vi "SMain.vi"() -> ()   [LabVIEW 2011] (continued)
          n194 = Equal?(x=w388, y="TRUE") -> ()  [unwired: 1 out]
          n195 = Equal?(x=w385, y="TRUE") -> (x = y?=w384:bool)
          n196 = local write "打印模式"(w347) -> ()
          n197 = case shown="\"N5224A\"" w396 {
            tunnel: [0 1 2] -> w395
            frame "E5071C", Default {
            }
            frame "N5230A(C)" {
            }
            frame "N5224A" {
            }
          }
          n198 = case shown="\"Dev3\"" w392 {
            tunnel: [0 1 2] -> w393
            frame "Dev1", Default {
            }
            frame "Dev2" {
            }
            frame "Dev3" {
            }
          }
          n199 = case shown="\"NI PCI-6509\", 默认" w394 {
            tunnel: [0 1] -> w350
            frame "NI PCI-6509", Default {
            }
            frame "LX MCU" {
            }
          }
          n200 = local write "Crosstalk  by Trace"(w372) -> ()
          n201 = local write "Local Database"(w384) -> ()
          n202 = local write "Dem 2X"(w368) -> ()
          n203 = local write "By Channel?"(w362) -> ()
          n204 = case shown="\"LUXSHARE - IIC\"" w344 {
            tunnel: [0 1] -> w346
            frame "RS232 - IIC", Default {
            }
            frame "LUXSHARE - IIC" {
            }
          }
          n205 = To Upper Case(1:w355) -> (0:w357:string)
          n206 = local write "RS232 I2C VISA"(w360) -> ()
          n207 = local write "VNA Model:"(w395) -> ()
          n208 = local write "Printer VISA"(w343) -> ()
          n209 = local write "DAQ  Model:"(w350) -> ()
          n210 = local write "DAQ Device"(w393) -> ()
          n211 = Equal?(x=w357, y="TRUE") -> (x = y?=w356:bool)
          n212 = local write "VISA COM"(w391) -> ()
          n213 = To Upper Case(1:w375) -> (0:w381:string)
          n214 = To Upper Case(1:w371) -> (0:w378:string)
          n215 = local write "upload"(w356) -> ()
          n216 = Equal?(x=w381, y="TRUE") -> (x = y?=w377:bool)
          n217 = Equal?(x=w378, y="TRUE") -> (x = y?=w376:bool)
          n218 = local write "Adaptor:"(w346) -> ()
          n219 = local write "Demo"(w377) -> ()
          n220 = local write "Manual"(w376) -> ()
          n221 = case shown="1" w350 {
            tunnel: [2 0] -> w352
            tunnel: [0 2] -> w351
            frame 0, Default {
            }
            frame 1 {
            }
          }
          n222 = disable-structure shown="禁用" {
            disable-tunnel: w356 -> [w401 _]
            frame Disabled {
              w402 = "Data UpLoad" ("项标识符")
              n223 = Current VI's Menubar() -> (w405:refnum<k9>)
              n224 = Get Menu Item Info(7:w402, 11:w405) -> (2:w403:string, 3:w404:refnum<k9>)  [unwired: 1 in, 5 out]
              n225 = Set Menu Item Info(6:w401, 7:w402, 9:TRUE ("已启用"), 10:w403, 11:w404) -> ()  [unwired: 2 in, 2 out]
            }
            frame Enabled {
            }
          }
          n226 = property on="DAQ Device" class="Ring (严格)"("DisabledEnum"=w351) -> ()  [unwired: 2 in, 2 out]
          n227 = property on="VISA COM" class="VISAName"("DisabledEnum"=w352) -> ()  [unwired: 2 in, 2 out]
          n228 = To Upper Case(1:w339) -> (0:w340:string)
          n229 = Equal?(x=w340, y="TRUE") -> (x = y?=w342:bool)
          n230 = local write "Use Counts?"(w342) -> ()
        }
      }
    }
    frame #4 {
      w441 = T8 {"Server"="", "DB"="", "PSW"="", "User"=""}  # DBSet
      n231 = call <vilib>:"Application Directory.vi"() -> ("Application Directory"=w498:path)
      n232 = Build Path(base path=w498, name or relative path="Database" ("名称或相对路径")) -> (appended path=w496:path)
      n233 = call <vilib>:"Application Directory.vi"() -> ("Application Directory"=w508:path)
      n234 = call <vilib>:"Application Directory.vi"() -> ("Application Directory"=w526:path)
      n235 = call <vilib>:"Check if File or Folder Exists.vi"("path"=w496) -> ("file or folder exists?"=w495:bool, "dup path"=w494:path)  [unwired: 8 in, 1 out]
      n236 = Build Path(base path=w526, name or relative path="EEPROM Code\\tempory_folder" ("名称或相对路径")) -> (appended path=w518:path)
      n237 = Build Path(base path=w508, name or relative path="Database" ("名称或相对路径")) -> (appended path=w506:path)
      n238 = case shown="假" w495 {
        tunnel: w494 -> [w555 w556]
        tunnel: [w554 w556] -> w493
        frame False {
          n239 = Create Folder(path (use dialog)=w555) -> (created path=w554:path)  [unwired: 2 in, 2 out]
        }
        frame True {
        }
      }
      n240 = call <vilib>:"Check if File or Folder Exists.vi"("path"=w518) -> ("file or folder exists?"=w517:bool, "dup path"=w516:path)  [unwired: 8 in, 1 out]
      n241 = call <vilib>:"Check if File or Folder Exists.vi"("path"=w506) -> ("file or folder exists?"=w505:bool, "dup path"=w504:path)  [unwired: 8 in, 1 out]
      n242 = case shown="假" w517 {
        tunnel: w516 -> [w579 w580]
        tunnel: [w578 w580] -> w515
        frame False {
          n243 = Create Folder(path (use dialog)=w579) -> (created path=w578:path)  [unwired: 2 in, 2 out]
        }
        frame True {
        }
      }
      n244 = case shown="假" w505 {
        tunnel: w504 -> [w574 w575]
        tunnel: [w573 w575] -> w503
        frame False {
          n245 = Create Folder(path (use dialog)=w574) -> (created path=w573:path)  [unwired: 2 in, 2 out]
        }
        frame True {
        }
      }
      n246 = Build Path(base path=w493, name or relative path="FigoConfig.xml" ("名称或相对路径")) -> (appended path=w491:path)
      n247 = call <vilib>:"Check if File or Folder Exists.vi"("path"=w491) -> ("file or folder exists?"=w490:bool, "dup path"=w466:path)  [unwired: 8 in, 1 out]
      n248 = call "deleteFolder_vna.vi"("input_path"=w515) -> ()  [unwired: 1 in]
      n249 = Build Path(base path=w503, name or relative path="DelayConfig.txt" ("名称或相对路径")) -> (appended path=w501:path)
      n250 = call <vilib>:"Check if File or Folder Exists.vi"("path"=w501) -> ("file or folder exists?"=w500:bool, "dup path"=w499:path)  [unwired: 8 in, 1 out]
      n251 = call <vilib>:"Application Directory.vi"() -> ("Application Directory"=w524:path)
      n252 = constructor class="CPLTSApplicationClass"() -> (reference out=w512:refnum<k24>)  [unwired: 3 in, 2 out]
      n253 = call "equipconfirm.vi"("path to XML document"=w466) -> ("确认结果"=w465:bool)
      n254 = Build Path(base path=w524, name or relative path="Database\\LabelList.xlsx" ("名称或相对路径")) -> (appended path=w522:path)
      n255 = call <vilib>:"Check if File or Folder Exists.vi"("path"=w522) -> ("error out"=w519:errorcluster, "file or folder exists?"=w521:bool, "dup path"=w520:path)  [unwired: 8 in]
      n256 = local read "打印模式"() -> (w511:enum16{"IT Print", "EE Print"})
      n257 = case shown="假" w465 {
        frame False {
          n258 = Quit LabVIEW(quit? (T)=TRUE ("退出？(T)")) -> ()
        }
        frame True {
        }
      }
      n259 = control-ref of="Test Status:"() -> (w422:refnum<vi>)
      n260 = case shown="真" w500 {
        tunnel: w499 -> [w561 w572]
        frame False {
          w557 = 100.0 ("写入延时（单位：ms）")
          w558 = 100.0 ("读取延时（单位：ms）")
          n261 = local write "读取延时（单位：ms）"(w558) -> ()
          n262 = global write "延时设置全局变量.vi" "写入延时"(w558) -> ()
          n263 = local write "Q写入延时（单位：ms）"(250.0 ("写入延时（单位：ms）")) -> ()
          n264 = local write "S写入延时（单位：ms）"(w557) -> ()
          n265 = global write "延时设置全局变量.vi" "写入延时"(w557) -> ()
          n266 = call-poly <vilib>:"Write To Spreadsheet File.vi"("2D data"=string[][] [["Q写入延时时间（ms）：", "250"], ["S写入延时时间（ms）：", "100"], ["读取延时时间（ms）：", "100"]], "file path (dialog if empty)"=w561) -> ()  [unwired: 6 in, 1 out]
        }
        frame True {
          n267 = call-poly <vilib>:"Read From Spreadsheet File.vi"("file path (dialog if empty)"=w572) -> ("all rows"=w571:string[][])  [unwired: 6 in, 4 out]
          n268 = Index Array(array=w571, index (col)=1 ("禁用的索引 (列)")) -> (element=w569:string[])  [unwired: 1 in]
          n269 = Index Array(array=w569, index #1=0 ("索引")) -> (element #1=w567:string, element #2=w565:string, element #3=w564:string)  [unwired: 2 in]
          n270 = Fract/Exp String To Number(string=w567) -> (number=w562:dbl)  [unwired: 3 in, 1 out]
          n271 = Fract/Exp String To Number(string=w564) -> (number=w566:dbl)  [unwired: 3 in, 1 out]
          n272 = Fract/Exp String To Number(string=w565) -> (number=w563:dbl)  [unwired: 3 in, 1 out]
          n273 = local write "Q写入延时（单位：ms）"(w562) -> ()
          n274 = global write "延时设置全局变量.vi" "写入延时"(w562) -> ()
          n275 = local write "S写入延时（单位：ms）"(w563) -> ()
          n276 = local write "读取延时（单位：ms）"(w566) -> ()
          n277 = global write "延时设置全局变量.vi" "读取延时"(w566) -> ()
        }
      }
      n278 = invoke class="CPLTSApplicationClass" method="ShowWindow"(reference=w512, "nCmdShow"="nCmdShow") -> (reference out=w514:refnum<k24>)  [unwired: 2 in, 3 out]
      n279 = case shown="\"IT Print\", 默认" w511 {
        frame "IT Print", Default {
          n280 = property on="MO:" class="Str"("Visible"=TRUE ("可见")) -> ()  [unwired: 2 in, 2 out]
        }
        frame "EE Print" {
          n281 = property on="MO:" class="Str"("Visible"=FALSE ("可见")) -> ()  [unwired: 2 in, 2 out]
        }
      }
      n282 = property on="属性节点" class="Str"(reference=w422, "Text.BGColor"=u32 16711680, "Text.TextColor"=u32 16448250) -> ()  [unwired: 1 in, 2 out]
      n283 = case shown="真" w490 {
        tunnel: w466 -> [_ w534]
        tunnel: [string[] ["net use \\\\172.200.20.86 Luxshare-ict /user:C040345", "\\\\172.20.20.86\\HuaweiData\\DataRoot\\XML", "net use \\\\172.20.20.113 mesuser /user:mesuser", "\\\\172.20.20.113\\emc\\HPTS\\VNA", "\\\\172.20.20.113\\emc\\HPTS\\SI", "false"] ("OutParaArray") w543] -> w489
        tunnel: [string[] ["false"] ("OutParaArray") w541] -> w472
        tunnel: ["A" ("node text") w537] -> w467
        tunnel: [string[] [] ("OutParaArray") w535] -> w451
        frame False {
        }
        frame True {
          w547 = "Mo" ("名称")
          w549 = "PN" ("名称")
          n284 = call "xmlConfigRead.vi"("path to XML document"=w534, "XPath expression"="//OtherPara/*") -> ("OutParaArray"=w541:string[])  [unwired: 2 out]
          n285 = call "xmlConfigRead.vi"("path to XML document"=w534, "XPath expression"="//UploadPara/*") -> ("OutParaArray"=w543:string[])  [unwired: 2 out]
          n286 = call "xmlConfigRead.vi"("path to XML document"=w534, "XPath expression"="//LastPartNo/*") -> ("OutParaVariant"=w551:variant)  [unwired: 2 out]
          n287 = call "xmlConfigRead.vi"("path to XML document"=w534, "XPath expression"="//LineID/Line/@Name") -> ("OutParaArray"=w532:string[])  [unwired: 2 out]
          n288 = call "xmlConfigRead.vi"("path to XML document"=w534, "XPath expression"="//DBSet/ConnectInfo/@*") -> ("OutParaArray"=w535:string[])  [unwired: 2 out]
          n289 = call "xmlConfigRead.vi"("path to XML document"=w534, "XPath expression"="//SystemList/CurrentNO/@Name") -> ("OutParaArray"=w539:string[])  [unwired: 2 out]
          n290 = Get Variant Attribute(Variant=w551, name=w549) -> (duplicate Variant=w552:variant, value=w550:variant)  [unwired: 2 in, 2 out]
          n291 = Get Variant Attribute(Variant=w552, name=w547) -> (value=w548:variant)  [unwired: 2 in, 3 out]
          n292 = property on="线别" class="Ring (严格)"("Strings []"=w532) -> ()  [unwired: 2 in, 2 out]
          n293 = Variant To Data(type=w547, Variant=w548) -> (data=w545:string)  [unwired: 1 in, 1 out]
          n294 = Variant To Data(type=w549, Variant=w550) -> (data=w546:string)  [unwired: 1 in, 1 out]
          n295 = property on="P/N:" class="Str"("Val(Sgnl)"=w546) -> ()  [unwired: 2 in, 2 out]
          n296 = local write "MO:"(w545) -> ()
          n297 = Index Array(array=w539, index=0 ("索引")) -> (element=w537:string)
        }
      }
      "SystemMode" <- w467
      n298 = case shown="假" w521 {
        tunnel: w520 -> [w584 _]
        tunnel: w519 -> [_ _]
        frame False {
          n299 = call <vilib>:"New Report.vi"("report type"=T16."Excel") -> ("report out"=w586:refnum<class "NI_report.lvclass">)  [unwired: 13 in, 1 out]
          n300 = call <vilib>:"Excel Get Worksheet.vi"("report in"=w586, "worksheet index (0)"=0) -> ("report out"=w588:refnum<class "NI_report.lvclass">, "error out"=w587:errorcluster)  [unwired: 12 in]
          n301 = Build Array(string[] ["料号", "日期类型", "年份起始位", "年份结束位", "周起始位", "周结束位", "月份起始位", "月份结束位", "天数起始位", "天数结束位", "流水号起始位", "流水号起始位"]) -> (w581:string[][])
          n302 = call-poly <vilib>:"Excel Easy Table.vi"("report in"=w588, "text data"=w581, "error in (no error)"=w587) -> ("report out"=w583:refnum<class "NI_report.lvclass">)  [unwired: 8 in, 4 out]
          n303 = call-dynamic "Save Report to File.vi"("report in"=w583, "report file path"=w584) -> ("report out"=w591:refnum<class "NI_report.lvclass">, "error out"=w590:errorcluster)  [unwired: 12 in]
          n304 = call-dynamic "Dispose Report.vi"("report in"=w591, "wait until printing completed? (T)"=TRUE, "error in (no error)"=w590) -> ()  [unwired: 12 in, 1 out]
        }
        frame True {
        }
      }
      n305 = local write "Excel?"(TRUE ("Excel?")) -> ()
      n306 = local write "upload"(TRUE ("upload")) -> ()
      n307 = invoke class="CPLTSApplicationClass" method="CloseAllFiles"(reference=w514) -> ()  [unwired: 2 in, 3 out]
      n308 = constructor class="LabelPrintHelper"() -> (reference out=→"PRINT":refnum<k24>)  [unwired: 3 in, 2 out]
      n309 = constructor class="MESDataServices"() -> (reference out=→"SN":refnum<k24>)  [unwired: 3 in, 2 out]
      n310 = Delete From Array(array=w451, length=4 ("长度")) -> (deleted portion=w442:string[], array with subset deleted=w450:string[])  [unwired: 1 in]
      n311 = Index Array(array=w450) -> (element #1=w449:string, element #2=w448:string, element #3=w446:string, element #4=w447:string)  [unwired: 4 in]
      n312 = global write "全局.vi" "print templete"(FALSE ("print templete")) -> ()
      n313 = call "DES.vi"("sourceData"=w446, "操作"=enum16{"DES_Encrypt", "DES_Decrypt"}."DES_Decrypt") -> ("加密后字符串"=w445:string)  [unwired: 8 in, 1 out]
      n314 = Index Array(array=w472, index #1=0 ("索引"), index #2=1 ("索引"), index #3=2 ("索引"), index #4=3 ("索引")) -> (element #1=w469:string, element #2=w462:string, element #3=w458:string, element #4=w453:string)
      n315 = Decimal String To Number(string=w453) -> (number=→"startSN":i32)  [unwired: 2 in, 1 out]
      n316 = Bundle By Name(cluster=w441, "Server"=w449, "DB"=w448, "PSW"=w445, "User"=w447) -> (→"DB1":T8)
      n317 = Decimal String To Number(string=w462) -> (number=w461:i32)  [unwired: 2 in, 1 out]
      n318 = Equal?(x=w469, y="true") -> (x = y?=→"ConvertStyle":bool)
      n319 = Index Array(array=w489, index #1=0 ("索引"), index #2=1 ("索引"), index #3=2 ("索引"), index #4=3 ("索引"), index #5=4 ("索引"), index #6=5 ("索引"), index #7=6 ("索引"), index #8=7 ("索引"), index #9=8 ("索引")) -> (element #1=→"NetCmd":string, element #2=→"NetPathHW":string, element #3=→"NetCmdCompress":string, element #4=w481:string, element #5=w480:string, element #6=w476:string, element #7=w428:string, element #8=→"NetTemppath":string, element #9=→"NetLocalpath":string)
      n320 = String To Path(string=w481) -> (path=→"NetPathCompress1":path)
      n321 = String To Path(string=w480) -> (path=→"NetPathCompress2":path)
      n322 = Equal?(x=w458, y="true") -> (x = y?=→"TestResultSave":bool)
      n323 = global write "全局.vi" "logsetting"(w461) -> ()
      n324 = Equal?(x=w476, y="true") -> (x = y?=→"AlarmDisplay":bool)
      n325 = Index Array(array=w442) -> (element #1=w440:string, element #2=w439:string, element #3=w437:string, element #4=w435:string)  [unwired: 4 in]
      n326 = call "DES.vi"("sourceData"=w437, "操作"=enum16{"DES_Encrypt", "DES_Decrypt"}."DES_Decrypt") -> ("加密后字符串"=w438:string)  [unwired: 8 in, 1 out]
      n327 = Equal?(x=w428, y="true") -> (x = y?=→"asychronus":bool)
      n328 = Bundle By Name(cluster=w441, "Server"=w440, "DB"=w439, "PSW"=w438, "User"=w435) -> (→"DB2":T8)
    }
    frame #5 {
      n329 = control-ref of="Test Status:"() -> (w593:refnum<vi>)
      n330 = global write "全局.vi" "Test Status"(w593) -> ()
      n331 = property on="Type" class="Ring (严格)"("Val(Sgnl)"=u16 0 ("值(信号)")) -> ()  [unwired: 2 in, 2 out]
      n332 = property on="Start Test" class="Bool"("BoolText.Text"="START TEST" ("布尔文本.文本")) -> ()  [unwired: 2 in, 2 out]
      n333 = local write "caliDataSelect"(FALSE ("caliDataSelect")) -> ()
    }
    frame #6 {
      n334 = while {
        tunnel: [w599] -> _
        stop <- w599 stop-if-true
        n335 = case shown="\"wait\", 默认" "State" {
          tunnel: [_ _ TRUE ("Stop") w1882] -> w599
          frame "test" {
            n336 = stacked-sequence {
              frame #0 {
                n337 = property on="Start Test" class="Bool"("DisabledEnum"=2) -> ()  [unwired: 2 in, 2 out]
                n338 = local write "proBar"(u8 0 ("proBar")) -> ()
                n339 = local write "preStation"("" ("preStation")) -> ()
                n340 = property on="preStation" class="Str"("Visible"=FALSE ("可见")) -> ()  [unwired: 2 in, 2 out]
                n341 = control-ref of="Test Status:"() -> (w601:refnum<vi>)
                n342 = property on="属性节点" class="Str"(reference=w601, "Text.BGColor"=u32 16448250, "Text.TextColor"=u32 0) -> ()  [unwired: 1 in, 2 out]
                n343 = property on="S/N:" class="Str"("DisabledEnum"=T17."Disabled and Grayed Out" ("禁用")) -> ()  [unwired: 2 in, 2 out]
                n344 = local write "strFSN 原始SN"("" ("strFSN 原始SN")) -> ()
                n345 = local write "Current Testing Label/当前测试条码"("") -> ()
                n346 = local write "midVar_time_date"(timestamp(3534465477 s since 1904-01-01) ("midVar_time_date")) -> ()
                n347 = local write "未经进制转换的sn(客户 jin zhi sn)"("" ("未经进制转换的sn(客户 jin zhi sn)")) -> ()
                n348 = local write "Test Status:"("" ("Test Status:")) -> ()
                n349 = local write "要烧录的DateCode"("" ("要烧录的DateCode")) -> ()
                n350 = local write "要烧录的时间和Sn"("" ("要烧录的时间和Sn")) -> ()
                "customer date" <- "" ("customer date")
                "Shi jin zhi sn" <- "" ("Shi jin zhi sn")
              }
              frame #1 {
                n351 = local read "Use Counts?"() -> (w619:bool)
                n352 = case shown="真" w619 {
                  tunnel: [TRUE w622] -> w618
                  frame False {
                  }
                  frame True {
                    n353 = local read "RS232 I2C Counts"() -> (w625:refnum<visa-resource-name>)
                    n354 = call "读取.vi"("RS232 I2C Counts"=w625) -> ("result"=w622:bool, "UseAge"=w623:i64, "Used"=w624:i64)  [unwired: 8 in]
                    n355 = local write "Used"(w624) -> ()
                    n356 = local write "UseAge"(w623) -> ()
                  }
                }
                n357 = local write "test time"(string[] [] ("test time")) -> ()
                n358 = case shown="真" w618 {
                  frame False {
                    # "测试版使用次数是否合格"
                    n359 = local read "UseAge"() -> (w630:i64)
                    n360 = local read "Used"() -> (w633:i64)
                    n361 = local write "Go"(FALSE ("Go")) -> ()
                    n362 = Number To Decimal String(number=w633) -> (decimal integer string=w632:string)  [unwired: 1 in]
                    n363 = Number To Decimal String(number=w630) -> (decimal integer string=w629:string)  [unwired: 1 in]
                    n364 = Concatenate Strings("测试板使用了", w632, "次,超过了最大使用寿命:" ("字符串"), w629, "不允许继续使用，请更换测试板后继续测试！" ("字符串"), "或者修改使用次数的动作失败！" ("字符串")) -> (w627:string)
                    n365 = One Button Dialog(message=w627) -> ()  [unwired: 1 in, 1 out]
                  }
                  frame True {
                    # "测试版使用次数是否合格"
                    n366 = local read "线别确认"() -> (w637:bool)
                    n367 = Not(x=w637) -> (.not. x?=w636:bool)
                    n368 = case shown="假" w636 {
                      frame False {
                        n369 = local read "DateCode8Value_0X30"() -> (w639:i32)
                        n370 = local read "打印模式"() -> (w642:enum16{"IT Print", "EE Print"})
                        n371 = local read "AutoSN"() -> (w643:bool)
                        n372 = local read "ConvertStyle"() -> (w641:bool)
                        n373 = Format Into String(initial string="当前datacode为:0X", w639) -> (resulting string=w638:string)  [unwired: 2 in, 1 out]
                        n374 = call "addStatus.vi"("msg"=w638) -> ()  [unwired: 10 in, 1 out]
                        n375 = case shown="假" w643 {
                          tunnel: w642 -> [_ w700]
                          tunnel: w641 -> [w653 w699]
                          tunnel: w639 -> [w652 w698]
                          frame False {
                            # "前站数据是否需要管控"
                            n376 = local read "S/N:"() -> (w650:string)
                            n377 = local read "P/N:"() -> (w645:string)
                            n378 = local read "DB1"() -> (w649:T8)
                            n379 = call "前站查询(T1).vi"("Station"="preStation", "Pre Check"="Pre Check", "PN"=w645, "DBSet"=w649, "SN"=w650) -> ("判定"=w648:bool)  [unwired: 6 in]
                            n380 = call "前站查询.vi"("DBSet"=w649, "SN"=w650) -> ("判定"=w647:bool)  [unwired: 9 in]
                            n381 = And(x=w647, y=w648) -> (x .and. y?=w646:bool)
                            n382 = case shown="真" w646 {
                              tunnel: w653 -> [_ w657]
                              tunnel: w652 -> [_ w656]
                              frame False {
                                n383 = One Button Dialog(message="前面有不良维修记录待处理，请进行处理后再测试" ("消息")) -> ()  [unwired: 1 in, 1 out]
                                n384 = local write "Go"(FALSE ("Go")) -> ()
                              }
                              frame True {
                                n385 = stacked-sequence {
                                tunnel: w657 -> [_ w665]
                                tunnel: w656 -> [_ w664]
                                frame #0 {
                                n386 = local read "DB1"() -> (w658:T8)
                                n387 = local read "LastSN"() -> (w662:string)
                                n388 = local read "S/N:"() -> (w661:string)
                                n389 = call "重测.vi"("Last SN"=w662, "DBSet"=w658, "SN"=w661) -> ("继续?"=→"继续?":bool, "重测原因"=→"重测原因":string)  [unwired: 6 in, 1 out]
                                }
                                frame #1 {
                                n390 = local read "继续?"() -> (w663:bool)
                                n391 = case shown="真" w663 {
                                tunnel: w665 -> [_ w677]
                                tunnel: w664 -> [_ w676]
                                frame False {
                                n392 = local write "Go"(FALSE ("Go")) -> ()
                                }
                                frame True {
                                # "20160919增加从labelprint表查询，理由：作业流程变更，第一站就打条码。"
                                # "针对重工已经打印标签\n的进行修改，从资讯\n数据库中查到SN对应\n的信息回来进行测试"
                                n393 = local read "DB1"() -> (w674:T8)
                                n394 = local read "P/N:"() -> (w696:string)
                                n395 = local read "Local Database"() -> (w668:bool)
                                n396 = local read "mid_str_labelType"() -> (w694:string)
                                n397 = local read "labelConfig"() -> (w693:string[])
                                n398 = local read "打印模式"() -> (w671:enum16{"IT Print", "EE Print"})
                                n399 = local read "校验信息"() -> (w673:T7)
                                n400 = Equal?(x=w671, y=enum16{"IT Print", "EE Print"}."EE Print") -> (x = y?=w669:bool)
                                n401 = Or(x=w668, y=w669) -> (x .or. y?=w667:bool)
                                n402 = local read "S/N:"() -> (w695:string)
                                "LastSN" <- w695
                                n403 = local read "mid_array_eep"() -> (w692:string[][])
                                n404 = call "精简框图4.vi"("P/N:"=w696, "mid_str_labelType"=w694, "DateCode8Value_0X30"=w676, "Convert Style"=w677, "LocalDataBase?"=w667, "labelConfig"=w693, "mid_array_eep"=w692, "SNKeep"="SN Keep", "S/N"=w695, "DBSet"=w674, "校验信息"=w673) -> ("show_date"=w681:timestamp, "要烧录的时间和Sn"=w691:string, "未经进制转换的sn(客户 jin zhi sn)"=w682:string, "要烧录的DateCode"=w690:string, "strFSN 原始 Customer sn"=w683:string, "输出的label内容"=w680:string, "Go"=w679:bool, "mid_array_temp_int"=w689:u8[][], "S/N:"=w688:string, "Customer Date"=w687:string, "shi jin zhi sn"=w686:string, "Report No."=w685:string, "Sample #"=w684:string)  [unwired: 4 in]
                                n405 = And(x=w679, y=TRUE) -> (x .and. y?=w678:bool)
                                n406 = local write "Go"(w678) -> ()
                                n407 = local write "midVar_time_date"(w681) -> ()
                                n408 = local write "strFSN 原始SN"(w683) -> ()
                                n409 = local write "未经进制转换的sn(客户 jin zhi sn)"(w682) -> ()
                                n410 = local write "要烧录的时间和Sn"(w691) -> ()
                                n411 = local write "要烧录的DateCode"(w690) -> ()
                                n412 = local write "Current Testing Label/当前测试条码"(w680) -> ()
                                n413 = local write "mid_array_temp_int"(w689) -> ()
                                n414 = local write "S/N:"(w688) -> ()
                                n415 = local write "customer date"(w687) -> ()
                                n416 = local write "Shi jin zhi sn"(w686) -> ()
                                n417 = local write "Report No."(w685) -> ()
                                n418 = local write "Sample #"(w684) -> ()
                                n419 = local write "midVar_str_SN"(w680) -> ()
                                }
                                }
                                }
                                }
                              }
                            }
                          }
                          frame True {
                            n420 = local write "重测原因"("firsttest" ("重测原因")) -> ()
                            n421 = case shown="\"IT Print\", 默认" w700 {
                              tunnel: w699 -> [w704 w733]
                              tunnel: w698 -> [w702 w727]
                              frame "IT Print", Default {
                                # "没有转进制的流水"
                                # "mid_array_temp_int 是展开后的烧录文件"
                                # "通过MIS获得Sn"
                                n422 = local read "MO:"() -> (w713:string)
                                n423 = local read "mid_str_labelType"() -> (w721:string)
                                n424 = local read "SN"() -> (w703:refnum<k24>)
                                n425 = local read "labelConfig"() -> (w720:string[])
                                n426 = local read "mid_array_eep"() -> (w719:string[][])
                                n427 = local read "P/N:"() -> (w722:string)
                                n428 = local read "校验信息"() -> (w701:T7)
                                n429 = call "精简框图3.vi"("P/N:"=w722, "mid_str_labelType"=w721, "DateCode8Value_0X30"=w702, "Convert Style"=w704, "新引用"=w703, "labelConfig"=w720, "mid_array_eep"=w719, "工单号"=w713, "校验信息"=w701) -> ("show_date"=w712:timestamp, "要烧录的时间和Sn"=→"要烧录的时间和Sn":string, "未经进制转换的sn(客户 jin zhi sn)"=w705:string, "要烧录的DateCode"=→"要烧录的DateCode":string, "strFSN 原始 Customer sn"=w708:string, "输出的label内容"=w711:string, "Go"=w714:bool, "mid_array_temp_int"=w718:u8[][], "S/N:"=w717:string, "Customer Date"=w707:string, "shi jin zhi sn"=w706:string, "Report No."=w716:string, "Sample #"=w715:string)  [unwired: 6 in]
                                "Current Testing Label/当前测试条码" <- w711
                                n430 = local write "mid_array_temp_int"(w718) -> ()
                                n431 = local write "S/N:"(w717) -> ()
                                n432 = local write "Report No."(w716) -> ()
                                n433 = local write "Sample #"(w715) -> ()
                                n434 = local write "midVar_str_SN"(w711) -> ()
                                n435 = local write "Go"(w714) -> ()
                                n436 = local write "midVar_time_date"(w712) -> ()
                                n437 = local write "未经进制转换的sn(客户 jin zhi sn)"(w705) -> ()
                                n438 = local write "strFSN 原始SN"(w708) -> ()
                                n439 = local write "customer date"(w707) -> ()
                                n440 = local write "Shi jin zhi sn"(w706) -> ()
                              }
                              frame "EE Print" {
                                n441 = local read "startSN"() -> (w724:i32)
                                n442 = control-ref of="Test Status:"() -> (w731:refnum<vi>)
                                n443 = local read "mid_str_labelType"() -> (w737:string)
                                n444 = local read "mid_str_snformat"() -> (w736:string)
                                n445 = local read "P/N:"() -> (w734:string)
                                n446 = local read "mid_array_eep"() -> (w732:string[][])
                                n447 = local read "校验信息"() -> (w723:T7)
                                n448 = property class="Str"(reference=w731) -> (reference out=w729:refnum<vi>, "Value"=w730:string)  [unwired: 1 in, 1 out]
                                n449 = call "精简框图1.vi"("mid_str_labelType"=w737, "mid_array_eep"=w732, "mid_str_snformat"=w736, "Convert Style"=w733, "DateCode8Value_0X30"=w727, "P/N"=w734, "Sart SN"=w724, "校验信息"=w723) -> ("LocalSN Generate Status"=w726:string, "midVar_time_date"=w738:timestamp, "midVar_str_SN"=w739:string, "mid_array_temp_int"=w740:u8[][], "S/N:"=w741:string, "Report No."=w742:string, "Sample #"=w743:string)  [unwired: 5 in]
                                n450 = Concatenate Strings(w730, "\n", w726) -> (w728:string)
                                n451 = local write "Go"(TRUE ("Go")) -> ()
                                n452 = local write "midVar_time_date"(w738) -> ()
                                n453 = local write "midVar_str_SN"(w739) -> ()
                                n454 = local write "mid_array_temp_int"(w740) -> ()
                                n455 = local write "S/N:"(w741) -> ()
                                n456 = local write "Report No."(w742) -> ()
                                n457 = local write "Sample #"(w743) -> ()
                                n458 = property class="Str"(reference=w729, "Value"=w728) -> ()  [unwired: 1 in, 2 out]
                              }
                            }
                          }
                        }
                      }
                      frame True {
                        n459 = local write "Go"(FALSE ("Go")) -> ()
                        n460 = One Button Dialog(message="线别未确认" ("消息")) -> ()  [unwired: 1 in, 1 out]
                      }
                    }
                  }
                }
              }
              frame #2 {
                n461 = local read "Go"() -> (w746:bool)
                n462 = case shown="真" w746 {
                  frame False {
                    w750 = 0
                    n463 = property on="S/N:" class="Str"("Key Focus"=TRUE ("键选中")) -> ()  [unwired: 2 in, 2 out]
                    n464 = local write "State"("wait" ("state")) -> ()
                    n465 = local write "S/N:"("") -> ()
                    n466 = property on="S/N:" class="Str"("DisabledEnum"=T17."Enabled" ("禁用")) -> ()  [unwired: 2 in, 2 out]
                    n467 = property on="Start Test" class="Bool"("DisabledEnum"=w750) -> ()  [unwired: 2 in, 2 out]
                    n468 = property on="Tab_Graph" class="TabCtl (严格)"("Value"=w750) -> ()  [unwired: 2 in, 2 out]
                  }
                  frame True {
                    n469 = local read "P/N:"() -> (w756:string)
                    n470 = local read "VNA Model:"() -> (w762:enum16{"E5071C", "N5230A(C)", "N5224A"})
                    n471 = local read "Spec _Col"() -> (w757:i32[])
                    n472 = control-ref of="Test Status:"() -> (w761:refnum<vi>)
                    n473 = local read "VNA VISA"() -> (w763:refnum<visa-resource-name>)
                    n474 = local read "S/N:"() -> (w760:string)
                    n475 = call "Sample name judge.vi"("Sample  Name:"=w756, "START input"=TRUE) -> ("START output"=w764:bool)
                    n476 = case shown="真" w764 {
                      tunnel: "DAQ Device" -> [_ w784]
                      tunnel: w763 -> [_ w783]
                      tunnel: w762 -> [_ w782]
                      tunnel: w761 -> [_ w781]
                      tunnel: w760 -> [_ w780]
                      tunnel: "Port Type" -> [_ w779]
                      tunnel: "Demo" -> [_ w778]
                      tunnel: w757 -> [_ w777]
                      tunnel: w756 -> [_ w776]
                      tunnel: "Manual" -> [_ w775]
                      tunnel: "VISA COM" -> [_ w774]
                      tunnel: "DAQ  Model:" -> [_ w773]
                      tunnel: "Crosstalk  by Trace" -> [_ w772]
                      frame False {
                        w771 = 0
                        n477 = property on="S/N:" class="Str"("Key Focus"=TRUE ("键选中")) -> ()  [unwired: 2 in, 2 out]
                        n478 = local write "State"("wait" ("state")) -> ()
                        n479 = local write "S/N:"("") -> ()
                        n480 = property on="Start Test" class="Bool"("DisabledEnum"=w771) -> ()  [unwired: 2 in, 2 out]
                        n481 = property on="S/N:" class="Str"("DisabledEnum"=T17."Enabled" ("禁用")) -> ()  [unwired: 2 in, 2 out]
                        n482 = property on="Tab_Graph" class="TabCtl (严格)"("Value"=w771) -> ()  [unwired: 2 in, 2 out]
                      }
                      frame True {
                        n483 = stacked-sequence {
                          seq-local: [_ _ _ _ _ _ _ _ _ _ w1439 _ _ _ _ _ _] -> [_ _ _ _ _ _ _ _ _ _ _ w1464 _ _ _ _ _]
                          tunnel: w784 -> [_ _ _ w925 w1066 w1161 _ _ _ _ _ w1483 _ _ _ _ _]
                          tunnel: w783 -> [_ _ _ w924 w1065 w1160 _ _ _ _ _ _ _ _ _ _ _]
                          tunnel: w782 -> [_ _ _ w923 w1064 w1159 _ _ _ _ _ _ _ _ _ _ _]
                          tunnel: w776 -> [_ _ w868 w922 w1063 w1158 _ _ _ _ _ _ _ _ _ _ _]
                          tunnel: w781 -> [_ _ w849 w921 w1062 w1157 _ _ w1281 w1345 w1441 w1481 w1531 _ w1727 _ _]
                          tunnel: w780 -> [_ _ w860 w920 w1061 w1156 _ _ _ _ _ _ _ _ _ _ _]
                          tunnel: w779 -> [_ _ _ w914 w1059 w1154 _ _ _ _ _ _ _ _ _ _ _]
                          tunnel: w778 -> [_ _ _ w904 w1049 w1144 _ w1261 _ w1343 _ w1476 _ _ w1722 w1778 _]
                          tunnel: w777 -> [_ _ _ w913 w1060 w1155 _ _ _ _ _ _ _ _ _ _ _]
                          tunnel: w775 -> [_ _ _ w903 w1048 w1143 _ _ _ _ _ w1477 _ _ _ _ _]
                          tunnel: w774 -> [_ _ _ w909 w1055 w1149 _ _ _ _ _ w1474 _ _ _ _ _]
                          tunnel: w773 -> [_ _ _ w908 w1054 w1148 _ _ _ _ _ w1473 _ _ _ _ _]
                          tunnel: w772 -> [_ _ w846 _ w1052 w1147 _ _ _ _ _ _ _ _ _ _ _]
                          frame #0 {
                            n484 = call <vilib>:"Application Directory.vi"() -> ("Application Directory"=w800:path)
                            n485 = Build Path(base path=w800, name or relative path="Database\\yellowLabelPN.txt" ("名称或相对路径")) -> (appended path=w798:path)
                            n486 = call <vilib>:"Check if File or Folder Exists.vi"("path"=w798) -> ("error out"=w795:errorcluster, "file or folder exists?"=w797:bool, "dup path"=w796:path)  [unwired: 8 in]
                            n487 = case shown="假" w797 {
                              tunnel: w796 -> [w807 w813]
                              tunnel: [w806 w814] -> _
                              tunnel: w795 -> [w805 w814]
                              tunnel: [w804 w813] -> w788
                              frame False {
                                n488 = stacked-sequence {
                                tunnel: w807 -> [w811 w812]
                                tunnel: [w810 _] -> w806
                                tunnel: w805 -> [w809 _]
                                tunnel: [_ w812] -> w804
                                frame #0 {
                                n489 = Write to Text File(file (use dialog)=w811, text="LR44" ("文本"), error in=w809) -> (error out=w810:errorcluster)  [unwired: 1 in, 2 out]
                                }
                                frame #1 {
                                }
                                }
                              }
                              frame True {
                              }
                            }
                            n490 = call-poly <vilib>:"Read From Spreadsheet File.vi"("file path (dialog if empty)"=w788) -> ("all rows"=w794:string[][])  [unwired: 6 in, 4 out]
                            n491 = Index Array(array=w794, index (col) #1=0 ("禁用的索引 (列)"), index (col) #2=1 ("索引 (列)")) -> (element #1=w792:string[], element #2=w786:string[])  [unwired: 2 in]
                            n492 = local read "P/N:"() -> (w791:string)
                            n493 = Search 1D Array(1D array=w792, element=w791) -> (index of element=w785:i32)  [unwired: 1 in]
                            n494 = Not Equal?(x=w785, y=-1) -> (x != y?=w789:bool)
                            n495 = case shown="真" w789 {
                              tunnel: w786 -> [_ w803]
                              tunnel: w785 -> [_ w802]
                              frame False {
                              }
                              frame True {
                                n496 = Index Array(array=w803, index=w802) -> (element=w801:string)
                                n497 = call "yellowLabelDialog.vi"("图片路径"=w801) -> ()  [unwired: 11 in]
                              }
                            }
                          }
                          frame #1 {
                            w819 = 8 ("y")
                            n498 = disable-structure shown="禁用" {
                              frame Disabled {
                                n499 = local read "Diff Test Item Name"() -> (w823:string[])
                                n500 = call "Divide Test Items.vi"("Test Item Name"=w823) -> ()  [unwired: 9 in, 2 out]
                              }
                              frame Enabled {
                              }
                            }
                            n501 = local read "S-Para Item List"() -> (w815:string[])
                            n502 = local write "db_ResultString"("") -> ()
                            n503 = Array Size(array=w815) -> (size(s)=w820:i32)
                            n504 = local read "Test Graph"() -> (w818:refnum<vi>[])
                            n505 = local read "Empty"() -> (w817:cluster{"Horz Time array":dbl[], "Y":dbl[]}[])
                            n506 = Less Or Equal?(x=w820, y=w819) -> (x <= y?=w821:bool)
                            n507 = Select(t=w820, s=w821, f=w819) -> (s? t:f=w822:i32)
                            n508 = for {
                              tunnel: w818 -> [w829] mode=indexing
                              tunnel: w817 -> [w828]
                              tunnel: w822 -> [w825]
                              tunnel: w815 -> [w827]
                              i -> [w824]
                              n509 = Index Array(array=w827, index=w824) -> (element=w826:string)
                              n510 = Less?(x=w824, y=w825) -> (x < y?=w830:bool)
                              n511 = case shown="假" w830 {
                                tunnel: w829 -> [w832 w836]
                                tunnel: w828 -> [w831 w835]
                                tunnel: w826 -> [_ w834]
                                frame False {
                                n512 = property class="XYGraph (严格)"(reference=w832, "Value"=w831, "Caption.Visible"=FALSE ("标题.可见")) -> ()  [unwired: 1 in, 2 out]
                                }
                                frame True {
                                n513 = property class="XYGraph (严格)"(reference=w836, "Value"=w835, "Caption.Visible"=TRUE ("标题.可见"), "Caption.Text"=w834) -> ()  [unwired: 1 in, 2 out]
                                }
                              }
                            }
                          }
                          frame #2 {
                            w841 = FALSE ("Urgent Stop")
                            w864 = 8 ("y")
                            n514 = stacked-sequence {
                              frame #0 {
                                n515 = local write "db_VNA"("" ("db_VNA")) -> ()
                              }
                              frame #1 {
                                w876 = ";" ("字符串")
                                n516 = local read "P/N:"() -> (w877:string)
                                n517 = local read "S/N:"() -> (w878:string)
                                n518 = Concatenate Strings(w877, w876, w878, w876) -> (w879:string)
                                n519 = local write "db_VNA"(w879) -> ()
                              }
                            }
                            n520 = local read "Dem 2X"() -> (w842:bool)
                            n521 = local read "S-Para Item List"() -> (w840:string[])
                            n522 = local read "2x equalize"() -> (w839:bool)
                            n523 = Bundle("Urgent Stop"=FALSE, "Crosstalk  by Trace"=w846, "Dem 2X"=w842, "2x equalize"=w839) -> (→"Option":T20)  [unwired: 1 in]
                            n524 = stacked-sequence {
                              tunnel: w849 -> [w894 w899]
                              tunnel: w868 -> [_ w898]
                              tunnel: w860 -> [_ w897]
                              frame #0 {
                                w895 = u16 1 items=["Normal Input", "Start", "Product Inf", "End"] ("Summary Method")
                                n525 = call "Summary Generating.vi"("Summary Method"=w895, "Status String"=w894) -> ()  [unwired: 26 in]
                              }
                              frame #1 {
                                w900 = u16 2 items=["Normal Input", "Start", "Product Inf", "End"] ("Summary Method")
                                n526 = local read "Length"() -> (w896:string)
                                n527 = call "Summary Generating.vi"("Summary Method"=w900, "Status String"=w899, "Sample S/N:"=w897, "Sample PN:"=w898, "Length(mm)"=w896) -> ()  [unwired: 23 in]
                              }
                            }
                            n528 = local read "Test Graph"() -> (w850:refnum<vi>[])
                            n529 = control-ref of="Tab_Graph"() -> (w851:refnum<vi>)
                            n530 = control-ref of="db_ResultString"() -> (w844:refnum<vi>)
                            n531 = Array Size(array=w840) -> (size(s)=w862:i32)
                            "S Item Size" <- w862
                            n532 = Get Date/Time In Seconds() -> (seconds since 1Jan1904=→"Start Time":timestamp)
                            n533 = Bundle("Tab_Graph"=w851, "Test Graph"=w850, "Test Status:"=w849, "db_ResultString"=w844) -> (→"Reference":T5)  [unwired: 1 in]
                            n534 = local write "Urgent Stop"(w841) -> ()
                            n535 = global write "全局.vi" "manual stop"(w841) -> ()
                            n536 = Get Date/Time In Seconds() -> (seconds since 1Jan1904=→"start":timestamp)
                            n537 = local read "TDR Test Item Name"() -> (w858:string[])
                            n538 = property on="Urgent Stop" class="Bool (严格)"("DisabledEnum"=0 ("索引")) -> ()  [unwired: 2 in, 2 out]
                            n539 = local read "S-para Pair Name"() -> (w874:string[])
                            n540 = property on="Start Test" class="Bool"("DisabledEnum"=2) -> ()  [unwired: 2 in, 2 out]
                            n541 = local read "NEXT Pair Name"() -> (w872:string[])
                            n542 = local read "FEXT Pair Name"() -> (w870:string[])
                            n543 = local read "Test Graph"() -> (w866:refnum<vi>[])
                            n544 = Array Size(array=w870) -> (size(s)=→"F-Pair Loop":i32)
                            n545 = Array Size(array=w872) -> (size(s)=→"N-Pair Loop":i32)
                            n546 = Array Size(array=w874) -> (size(s)=→"S-Pair Loop":i32)
                            n547 = Array Size(array=w858) -> (size(s)=→"T Item Size":i32)
                            n548 = Less Or Equal?(x=w862, y=w864) -> (x <= y?=w865:bool)
                            n549 = local read "Empty"() -> (w861:cluster{"Horz Time array":dbl[], "Y":dbl[]}[])
                            n550 = Select(t=w862, s=w865, f=w864) -> (s? t:f=w863:i32)
                            n551 = for {
                              tunnel: w866 -> [w885] mode=indexing
                              tunnel: w861 -> [w884]
                              tunnel: w863 -> [w881]
                              tunnel: w840 -> [w883]
                              i -> [w880]
                              n552 = Index Array(array=w883, index=w880) -> (element=w882:string)
                              n553 = Less?(x=w880, y=w881) -> (x < y?=w886:bool)
                              n554 = case shown="假" w886 {
                                tunnel: w885 -> [w888 w892]
                                tunnel: w884 -> [w887 w891]
                                tunnel: w882 -> [_ w890]
                                frame False {
                                n555 = property class="XYGraph (严格)"(reference=w888, "Value"=w887, "Caption.Visible"=FALSE ("标题.可见")) -> ()  [unwired: 1 in, 2 out]
                                }
                                frame True {
                                n556 = property class="XYGraph (严格)"(reference=w892, "Value"=w891, "Caption.Visible"=TRUE ("标题.可见"), "Caption.Text"=w890) -> ()  [unwired: 1 in, 2 out]
                                }
                              }
                            }
                            n557 = property on="Result" class="Str"("Visible"=TRUE ("可见"), "Text.Text"="Testing..." ("文本.文本"), "Text.TextColor"=u32 16860, "Text.FontSize"=u32 40 ("文本.字体:字号"), "Blinking"=FALSE ("闪烁")) -> ()  [unwired: 2 in, 2 out]
                          }
                          frame #3 {
                            n558 = local read "T Item Size"() -> (w918:i32)
                            n559 = local read "S Item Size"() -> (w919:i32)
                            n560 = local read "ILD Spec No"() -> (w911:i32)
                            n561 = local read "Urgent Stop"() -> (w907:bool)
                            n562 = Greater Than 0?(x=w918) -> (x > 0?=w917:bool)
                            n563 = Greater Than 0?(x=w919) -> (x > 0?=w916:bool)
                            n564 = Bundle("Demo"=w904, "Manual"=w903, "Urgent Stop"="Urgent Stop") -> (w906:T21)  [unwired: 1 in]
                            n565 = Or(x=w917, y=w916) -> (x .or. y?=w915:bool)
                            "Thru?" <- w915
                            n566 = case shown="真" w915 {
                              tunnel: w925 -> [_ w947]
                              tunnel: w924 -> [_ w946]
                              tunnel: w923 -> [_ w945]
                              tunnel: w922 -> [_ w944]
                              tunnel: w921 -> [_ w943]
                              tunnel: w904 -> [_ w942]
                              tunnel: w920 -> [_ w941]
                              tunnel: w914 -> [_ w940]
                              tunnel: w913 -> [_ w939]
                              tunnel: [TRUE ("Total Reult") w938] -> w912
                              tunnel: w911 -> [_ w937]
                              tunnel: ["" ("String data") w936] -> w910
                              tunnel: w909 -> [_ w935]
                              tunnel: w908 -> [_ w934]
                              tunnel: w907 -> [_ w933]
                              tunnel: w906 -> [_ w932]
                              tunnel: [bool[] [TRUE] ("Testing Results") w931] -> w902
                              tunnel: [string[] [] ("S-Para Item List") w930] -> w901
                              frame False {
                              }
                              frame True {
                                n567 = stacked-sequence {
                                seq-local: [_ _ _ w1007 _] -> [_ _ _ _ w1033]
                                tunnel: w947 -> [w959 _ _ _ _]
                                tunnel: w946 -> [_ _ _ w1022 _]
                                tunnel: w945 -> [_ _ _ w1012 _]
                                tunnel: w944 -> [_ _ _ w996 _]
                                tunnel: w943 -> [w969 _ _ _ _]
                                tunnel: w942 -> [_ _ _ _ _]
                                tunnel: w941 -> [_ _ _ w995 _]
                                tunnel: w940 -> [_ _ _ w1015 _]
                                tunnel: w939 -> [_ _ _ _ _]
                                tunnel: [_ _ _ w1007 _] -> w938
                                tunnel: w937 -> [_ _ _ w1014 _]
                                tunnel: [_ _ _ w1011 _] -> w936
                                tunnel: w935 -> [_ _ _ w1010 _]
                                tunnel: w934 -> [_ _ _ w987 _]
                                tunnel: w933 -> [_ _ _ _ _]
                                tunnel: w932 -> [_ _ _ w1004 _]
                                tunnel: [_ _ _ w999 _] -> w931
                                tunnel: [_ _ _ w994 _] -> w930
                                frame #0 {
                                w968 = u16 0 items=["Normal Input", "Start", "Product Inf", "End"] ("Summary Method")
                                # "一定要选第6项，StepImpedance\n20160926"
                                n568 = local read "Switch array"() -> (w958:bool[][])
                                n569 = local read "Skew Spec(ps)"() -> (w954:i32)
                                n570 = Bundle("DAQ Device"=w959, "Switch array"=w958, 0) -> (→"Matrix In":T22)  [unwired: 1 in]
                                n571 = local read "CMP setting"() -> (w949:string)
                                n572 = Bundle("Start TimeNs"="Start TimeNs", "StopTimeNs"="StopTimeNs", "Data Points"="Data Points", "Compensation(ohm)"="Compensation(ohm)", "DataFormat"="DataFormat", "Impedance Filter"="Impedance Filter", "Filter Risetime(ps)"="Filter Risetime(ps)", "Impedance Spec String"="Impedance Spec String", "Skew Spec(ps)"=w954, "CMP setting"=w949) -> (→"TDR Setting":T12)  [unwired: 1 in]
                                n573 = call "Summary Generating.vi"("Summary Method"=w968, "Status String"=w969, "String 2"="S-parameter Testing....." ("Test Status:")) -> ()  [unwired: 25 in]
                                n574 = Format Date/Time String(time format string (%c)="%Y/%m/%d %H:%M:%S" ("时间格式字符串(%c)")) -> (date/time string=w953:string)  [unwired: 2 in]
                                n575 = call <vilib>:"Trim Whitespace.vi"("string"=w953) -> ("trimmed string"=w951:string)  [unwired: 1 in]
                                n576 = Build Array(w951) -> (w950:string[])
                                n577 = local write "test time"(w950) -> ()
                                }
                                frame #1 {
                                n578 = case shown="真" "Impedance Filter 2" {
                                selector: "Impedance Filter 2" -> [_ w977]
                                frame False {
                                n579 = local read "TDR Setting"() -> (→"TDR Setting 2":T12)
                                }
                                frame True {
                                n580 = local read "DataFormat"() -> (w978:i16)
                                n581 = local read "Skew Spec(ps) 2"() -> (w974:i32)
                                n582 = Bundle("Start TimeNs 2"="Start TimeNs 2", "StopTimeNs 2"="StopTimeNs 2", "Data Points 2"="Data Points 2", "Compensation(ohm) 2"="Compensation(ohm) 2", "DataFormat"=w978, w977, "Filter Risetime(ps) 2"="Filter Risetime(ps) 2", "Impedance Spec String 2"="Impedance Spec String 2", "Skew Spec(ps) 2"=w974, "") -> (w973:T23)  [unwired: 1 in]
                                n583 = local write "TDR Setting 2"(w973) -> ()
                                }
                                }
                                }
                                frame #2 {
                                n584 = local read "TDR Setting 2"() -> (w984:T10)
                                n585 = local read "TDR Setting"() -> (w985:T12)
                                n586 = Build Array(w985, w984) -> (→"TDR setting array":T6)
                                }
                                frame #3 {
                                n587 = local read "S-Para Item List"() -> (w1009:string[])
                                n588 = local read "TDR Test Item Name"() -> (w1008:string[])
                                n589 = local read "S-para Pair Name"() -> (w993:string[])
                                n590 = local read "Length"() -> (w992:string)
                                n591 = local read "Diff Test Item Name"() -> (w991:string[])
                                n592 = local read "Diff Test Item smooth"() -> (w990:string[])
                                n593 = local read "smooth point"() -> (w989:i32)
                                n594 = local read "limitSpec"() -> (w986:string[][])
                                n595 = Insert Into Array(array=w1009, new element=w1008) -> (w994:string[])  [unwired: 1 in]
                                "itemList" <- w994
                                n596 = Bundle By Name(cluster="Information In", "Sample PN:"=w996, "SampleSN:"=w995, "Sparam Test Item"=w994, "S-para Pair Name"=w993, "Length"=w992, "Diff Test Item Name"=w991, "Diff Test Item Name smooth"=w990, "smooth point"=w989, "limitSpec"=w986) -> (w988:T4)
                                n597 = local read "Reference"() -> (w1003:T5)
                                n598 = local read "proBar_ref"() -> (w1000:refnum<vi>)
                                n599 = local read "TDR setting array"() -> (w998:T6)
                                n600 = local read "Option"() -> (w1005:T11)
                                n601 = local read "Matrix In"() -> (w1017:T13)
                                n602 = local read "2X IL"() -> (w1006:dbl[])
                                n603 = call "Sparameter Testing.vi"("VNA Model:"=w1012, "VNA VISA"=w1022, "Port Type"=w1015, "Reference"=w1003, "VISA COM"=w1010, "Information In"=w988, "TDR setting array"=w998, "Mode(Demo,Manual)"=w1004, "DAQ  Model:"=w987, "S4P Data Type"=enum16{"THRU", "NEXT", "FEXT"}."THRU", "Matrix  In"=w1017, "ILDSpec"=w1014, "Option"=w1005, "MulChannel?"="By Channel?", "2X Thru"=w1006, "proBar_ref"=w1000) -> ("String data"=w1011:string, "Basic Path"=→"original Path":path, "Frequency(Hz)"=→"Frequency(Hz)":dbl[], "Data Out"=→"Data Out":dbl[][][], "Testing Results"=w999:bool[], "Total Reult"=w1007:bool, "TXT Data Path"=→"TXT Data Path":path, "Items Result"=→"Items Result":string[], "S4P Data Path"=→"S4P Data Path":path)  [unwired: 2 in, 1 out]
                                }
                                frame #4 {
                                n604 = local read "S-Para Item List"() -> (w1038:string[])
                                n605 = local read "TDR Test Item Name"() -> (w1023:string[])
                                n606 = local read "Items Result"() -> (w1039:string[])
                                n607 = Array Size(array=w1038) -> (size(s)=w1037:i32)
                                n608 = Split 1D Array(array=w1039, index=w1037) -> (first subarray=w1036:string[], second subarray=w1026:string[])
                                n609 = Search 1D Array(1D array=w1023, element="Pskew" ("元素")) -> (index of element=w1025:i32)  [unwired: 1 in]
                                n610 = Not Equal?(x=w1025, y=-1) -> (x != y?=w1027:bool)
                                n611 = case shown="真" w1027 {
                                tunnel: w1026 -> [w1040 w1044]
                                tunnel: w1025 -> [_ w1043]
                                tunnel: [w1040 w1041] -> w1024
                                frame False {
                                }
                                frame True {
                                n612 = Delete From Array(array=w1044, length=1 ("长度"), index=w1043) -> (array with subset deleted=w1041:string[])  [unwired: 1 out]
                                }
                                }
                                n613 = Select(t="PASS" ("字符串"), s=w1033, f="FAIL" ("字符串")) -> (s? t:f=w1031:string)
                                n614 = Insert Into Array(array=w1024, new element=w1036) -> (w1032:string[])  [unwired: 1 in]
                                n615 = Insert Into Array(array=w1032, new element=w1031) -> (w1030:string[])  [unwired: 1 in]
                                n616 = local write "Items Result"(w1030) -> ()
                                }
                                }
                              }
                            }
                            "SparaReult" <- w912
                            "Thru String data" <- w910
                            "SparaReults" <- w902
                            "SparaLists" <- w901
                          }
                          frame #4 {
                            n617 = local read "Diff Test Item Name"() -> (w1058:string[])
                            n618 = local read "Urgent Stop"() -> (w1051:bool)
                            n619 = local read "limitSpec"() -> (w1045:string[][])
                            n620 = local read "NEXT Pair Name"() -> (w1068:string[])
                            n621 = Bundle("Demo"=w1049, "Manual"=w1048, "Urgent Stop"=w1051) -> (w1050:T21)  [unwired: 1 in]
                            n622 = Search 1D Array(1D array=w1058, element="NEXT" ("元素")) -> (index of element=w1067:i32)  [unwired: 1 in]
                            n623 = local read "Urgent Stop"() -> (w1053:bool)
                            n624 = Not Equal?(x=w1067, y=-1) -> (x != y?=w1069:bool)
                            "NEXT?" <- w1069
                            n625 = case shown="真" w1069 {
                              tunnel: w1068 -> [_ w1095]
                              tunnel: w1045 -> [_ w1094]
                              tunnel: w1060 -> [_ w1093]
                              tunnel: w1067 -> [_ w1092]
                              tunnel: w1066 -> [_ w1091]
                              tunnel: w1065 -> [_ w1090]
                              tunnel: w1064 -> [_ w1089]
                              tunnel: w1063 -> [_ w1088]
                              tunnel: w1062 -> [_ w1087]
                              tunnel: w1061 -> [_ w1086]